vi "Interfaz_Gardenias.vi"() -> ()   [LabVIEW 2020]
uses:
  <vilib>/Instr/_visa.llb/VISA Configure Serial Port (Instr).vi
panel:
  in  "VISA resource name":refnum<visa-resource-name>
  out "Valor Tanque":dbl
  out "Valores actuales":string
  out "Humedad relativa":dbl
  out "Humedad tierra":dbl
  out "Temperatura":dbl
  out "Tanque":dbl
  out "Iteraciones":i32
  out "Tank":dbl(slide) scale=0.0..10.0
  out "Nivel Alto":bool
  out "Nivel Medio":bool
  out "Nivel Bajo":bool
  out "Array":string[](array[string])
  in  "stop":bool
  # "Proyecto terrario"
  # "Gardenia"
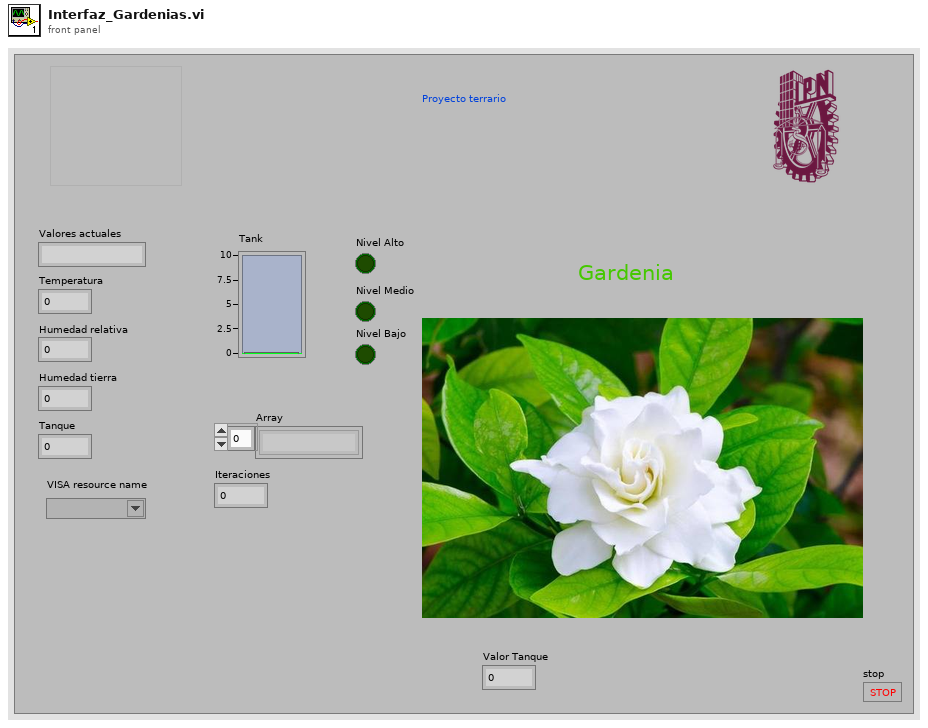
[diagram p1: front panel]
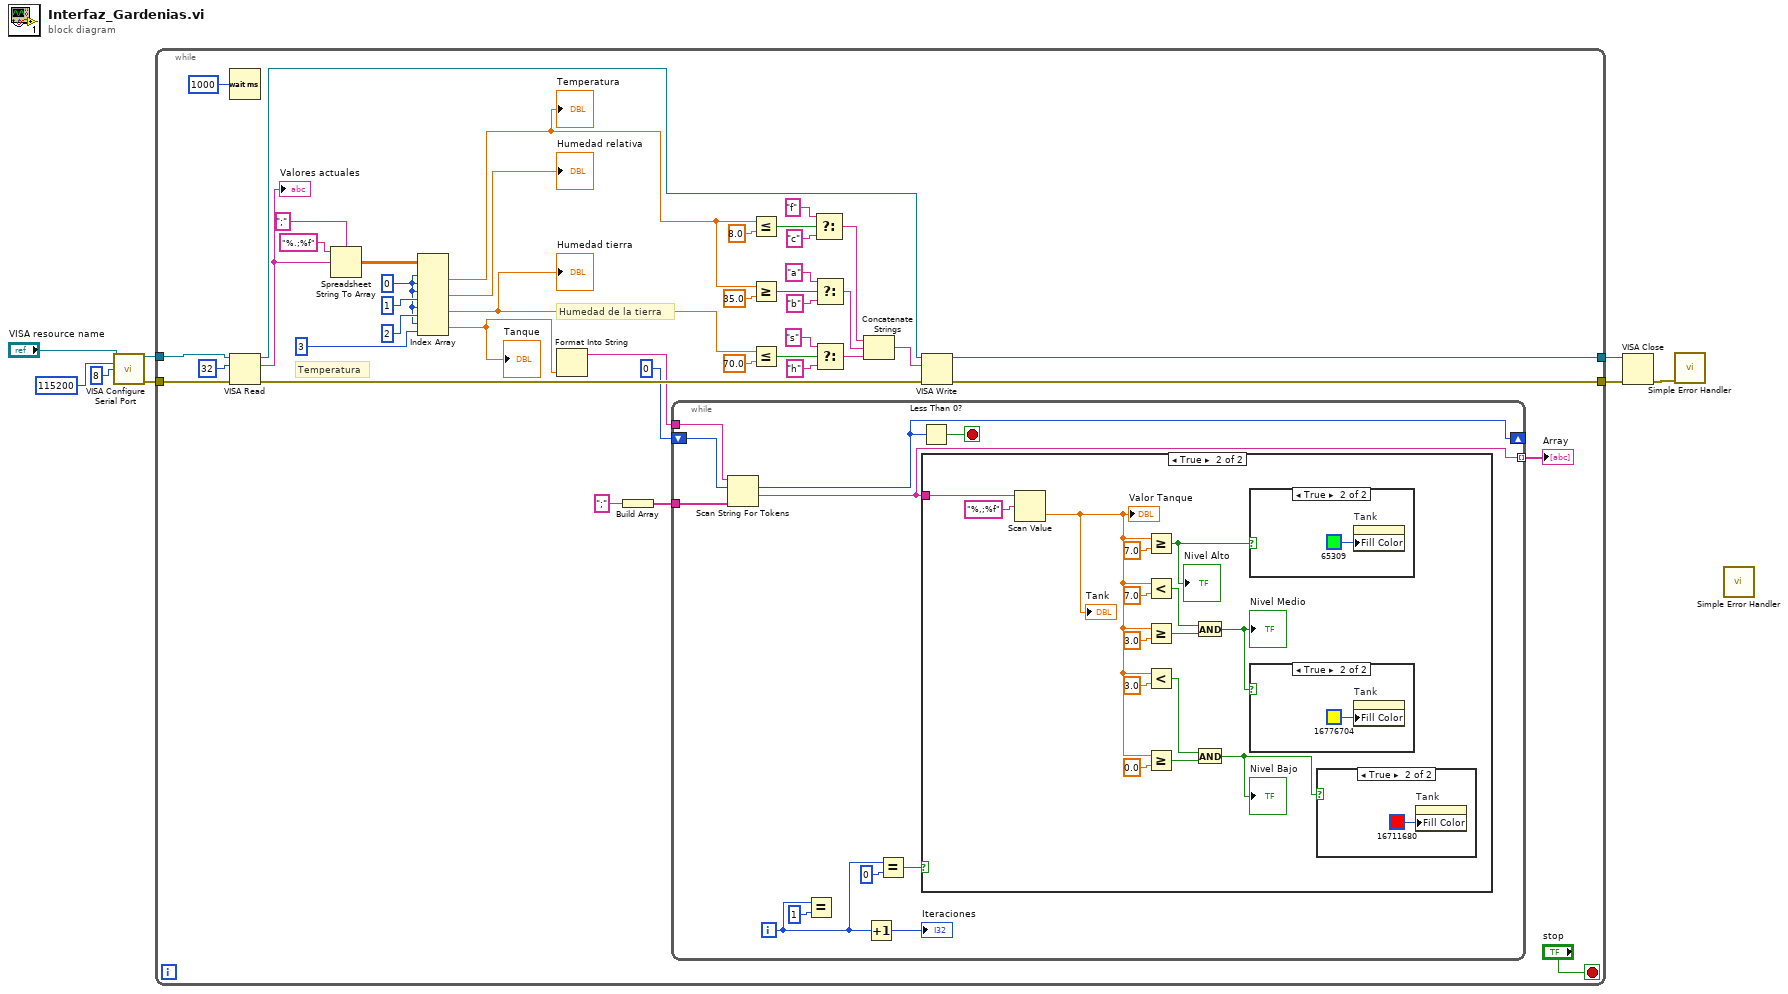
[diagram p0: block diagram]
diagram:
  n1 = call-poly "VISA Configure Serial Port"("VISA resource name"="VISA resource name", "baud rate (9600)"=u32 115200, "data bits (8)"=u16 8) -> ("VISA resource name out"=w7:refnum<visa-resource-name>, "error out"=w6:errorcluster)  [unwired: 11 in]
  n2 = while {
    tunnel: w7 -> [w10]
    tunnel: w6 -> [w9]
    tunnel: [w38] -> w3
    tunnel: [w37] -> w2
    stop <- "stop" stop-if-true
    w42 = 0 ("index (row)")
    # "Humedad de la tierra"
    # "Temperatura"
    n3 = Wait (ms)(milliseconds to wait=u32 1000) -> ()  [unwired: 1 out]
    n4 = VISA Read(VISA resource name=w10, byte count=u32 32, error in (no error)=w9) -> (VISA resource name out=w39:refnum<visa-resource-name>, read buffer=w44:string, error out=w40:errorcluster)  [unwired: 1 out]
    "Valores actuales" <- w44
    n5 = Spreadsheet String To Array(delimiter (Tab)=";", format string="%.;%f", spreadsheet string=w44) -> (array=w46:dbl[][])  [unwired: 1 in]
    n6 = Index Array "Index Array"(array=w46, index (row) #1=w42, index (col) #1=w42, index (row) #2=w42, index (col) #2=1 ("disabled index (col)"), index (row) #3=w42, index (col) #3=2 ("disabled index (col)"), index (row) #4=w42, index (col) #4=3 ("disabled index (col)")) -> (element #1=w31:dbl, element #2=→"Humedad relativa":dbl, element #3=w20:dbl, element #4=w12:dbl)
    "Humedad tierra" <- w20
    "Temperatura" <- w31
    "Tanque" <- w12
    n7 = Format Into String(w12) -> (resulting string=w13:string)  [unwired: 3 in, 1 out]
    n8 = Build Array(";") -> (w16:string[])
    n9 = while {
      shift-right: [w53] -> _
      shift-left: u32 0 ("milliseconds to wait") -> [w54]
      tunnel: w13 -> [w61]
      tunnel: w16 -> [w60]
      tunnel: [w52] -> w15 mode=indexing
      i -> [w57]
      stop <- w56 stop-if-true
      n10 = Scan String For Tokens(6:w60, 8:w54, 9:w61) -> (1:w52:string, 2:w53:i32)  [unwired: 3 in, 2 out]
      n11 = Equal?(x=w57, y=u32 1 ("milliseconds to wait")) -> ()  [unwired: 1 out]
      n12 = Increment(x=w57) -> (x+1=→"Iteraciones":i32)
      n13 = Equal?(x=w57, y=u32 0 ("milliseconds to wait")) -> (x = y?=w51:bool)
      n14 = Less Than 0?(x=w53) -> (x < 0?=w56:bool)
      n15 = case shown="True" w51 {
        tunnel: w52 -> [_ w75]
        frame False {
        }
        frame True {
          n16 = Scan Value(string=w75, format string="%,;%f") -> (value=w65:dbl)  [unwired: 1 in, 1 out]
          "Valor Tanque" <- w65
          "Tank" <- w65
          n17 = Greater Or Equal?(x=w65, y=7.0) -> (x >= y?=w64:bool)
          "Nivel Alto" <- w64
          n18 = Less?(x=w65, y=7.0) -> (x < y?=w71:bool)
          n19 = Greater Or Equal?(x=w65, y=3.0) -> (x >= y?=w73:bool)
          n20 = Less?(x=w65, y=3.0) -> (x < y?=w67:bool)
          n21 = Greater Or Equal?(x=w65, y=0.0) -> (x >= y?=w66:bool)
          n22 = And(x=w71, y=w73) -> (x .and. y?=w63:bool)
          "Nivel Medio" <- w63
          n23 = And(x=w67, y=w66) -> (x .and. y?=w62:bool)
          "Nivel Bajo" <- w62
          n24 = case shown="True" w64 {
            frame False {
            }
            frame True {
              n25 = property on="Tank" class="Slide (strict)"("Fill Color"=u32 65309) -> ()  [unwired: 2 in, 2 out]
            }
          }
          n26 = case shown="True" w63 {
            frame False {
            }
            frame True {
              n27 = property on="Tank" class="Slide (strict)"("Fill Color"=u32 16776704) -> ()  [unwired: 2 in, 2 out]
            }
          }
          n28 = case shown="True" w62 {
            frame False {
            }
            frame True {
              n29 = property on="Tank" class="Slide (strict)"("Fill Color"=u32 16711680) -> ()  [unwired: 2 in, 2 out]
            }
          }
        }
      }
    }
    "Array" <- w15
    n30 = Less Or Equal?(x=w31, y=8.0) -> (x <= y?=w32:bool)
    n31 = Greater Or Equal?(x=w31, y=35.0) -> (x >= y?=w36:bool)
    n32 = Less Or Equal?(x=w20, y=70.0) -> (x <= y?=w24:bool)
    n33 = Select(t="f", s=w32, f="c") -> (s? t:f=w26:string)
    n34 = Select(t="a", s=w36, f="b") -> (s? t:f=w27:string)
    n35 = Select(t="s", s=w24, f="h") -> (s? t:f=w19:string)
    n36 = Concatenate Strings(w26, w27, w19) -> (w25:string)
    n37 = VISA Write(VISA resource name=w39, write buffer=w25, error in (no error)=w40) -> (VISA resource name out=w38:refnum<visa-resource-name>, error out=w37:errorcluster)  [unwired: 1 out]
  }
  n38 = VISA Close(VISA resource name=w3, error in (no error)=w2) -> (error out=w5:errorcluster)
  n39 = call <vilib>:"Simple Error Handler.vi"("error in (no error)"=w5) -> ()  [unwired: 4 in, 5 out]
  n40 = call <vilib>:"Simple Error Handler.vi"() -> ()  [unwired: 5 in, 5 out]
